vi "HFRR ADV v038.vi"() -> ()   [LabVIEW 2025] (continued)
        n794 = property on="Tab Control 5" class="TabCtl (strict)"("Value"=enum32{"OK", "NG"}."NG" ("Tab Control 5")) -> ()  [unwired: 2 in, 2 out]
      }
      frame True {
        n795 = property on="Accept & Save" class="Bool (strict)"("DisabledEnum"=T19."Enabled" ("Disabled")) -> ()  [unwired: 2 in, 2 out]
        n796 = property on="Tab Control 5" class="TabCtl (strict)"("Value"=enum32{"OK", "NG"}."OK" ("Tab Control 5")) -> ()  [unwired: 2 in, 2 out]
      }
    }
    n797 = local read "Quit"() -> (w735:bool)
  }
  n798 = while {
    shift-right: [w815] -> _
    shift-left: "Enum - Selector" -> [w816]
    stop <- w817 stop-if-true
    # "Auto Start Logic Loop"
    n799 = case shown="\"close\"" w816 {
      tunnel: [w820 w826 w853 w885 w915 Auto_Start_enum."Exit" ("Enum - Selector") Auto_Start_enum."Init" ("Enum - Selector")] -> w815
      frame "Init", Default {
        n800 = local read "Auto Start Test"() -> (w819:bool)
        n801 = Select(t=Auto_Start_enum."Humidity & Temperature On" ("Enum - Selector"), s=w819, f=Auto_Start_enum."Init") -> (s? t:f=w820:T15)
      }
      frame "Humidity & Temperature On" {
        n802 = stacked-sequence {
          tunnel: [_ _ _ _ _ _ Auto_Start_enum."Reach point" ("Enum - Selector")] -> w823
          frame #0 {
            w828 = T19."Disabled and Grayed Out" ("Disabled")
            w829 = TRUE ("Heater Button")
            n803 = property on="Humidity" class="Bool (strict)"("DisabledEnum"=w828) -> ()  [unwired: 2 in, 2 out]
            n804 = property on="Heater Button" class="Bool (strict)"("DisabledEnum"=w828) -> ()  [unwired: 2 in, 2 out]
            n805 = local write "Heater Button"(w829) -> ()
            n806 = local write "Humidity"(w829) -> ()
            n807 = property on="Heater Button" class="Bool (strict)"("Val(Sgnl)"=TRUE ("Value (Signaling)")) -> ()  [unwired: 2 in, 2 out]
          }
          frame #1 {
            n808 = Wait (ms)(milliseconds to wait=u32 3000) -> ()  [unwired: 1 out]
          }
          frame #2 {
            n809 = local read "Set Temp"() -> (w835:dbl)
            n810 = Number To Fractional String(number=w835, precision (6)=i16 2) -> (F-format string=w832:string)  [unwired: 2 in]
            n811 = Concatenate Strings("ST;" ("Command"), w832) -> (w833:string)
            n812 = local write "Due Write"(w833) -> ()
          }
          frame #3 {
            n813 = Wait (ms)(milliseconds to wait=u32 1500) -> ()  [unwired: 1 out]
          }
          frame #4 {
            (unwired) i16 2 ("precision (6)")
            n814 = local read "WriteHumidity"() -> (w837:string[])
            n815 = local read "Set Rh"() -> (w840:dbl)
            n816 = Number To Fractional String(number=w840) -> (F-format string=w841:string)  [unwired: 3 in]
            n817 = Concatenate Strings("M;" ("new element/subarray"), w841) -> (w842:string)
            n818 = Insert Into Array(array=w837, new element=w842) -> (w838:string[])  [unwired: 1 in]
            n819 = local write "WriteHumidity"(w838) -> ()
            n820 = local write "Due Write"("HE;1" ("Command")) -> ()
          }
          frame #5 {
            n821 = Wait (ms)(milliseconds to wait=u32 1500) -> ()  [unwired: 1 out]
          }
          frame #6 {
            w845 = TRUE ("Reach point temp")
            n822 = local write "Reach point Humidity"(w845) -> ()
            n823 = local write "Reach point temp"(w845) -> ()
          }
        }
        n824 = local read "Auto Start Test"() -> (w825:bool)
        n825 = Not(x=w825) -> (.not. x?=w824:bool)
        n826 = Select(t=Auto_Start_enum."close", s=w824, f=w823) -> (s? t:f=w826:T15)
      }
      frame "Reach point" {
        w854 = TRUE ("PAUSE")
        w862 = 1.0 ("y")
        w865 = 1.0 ("y")
        n827 = local read "Set Temp"() -> (w847:dbl)
        n828 = local read "Set Humidity:"() -> (w861:dbl)
        n829 = local read "Humidity ( %RH )"() -> (w866:dbl)
        n830 = Add(x=w847, y=w865) -> (x+y=w864:dbl)
        n831 = Subtract(x=w847, y=w865) -> (x-y=w863:dbl)
        n832 = Add(x=w861, y=w862) -> (x+y=w860:dbl)
        n833 = Subtract(x=w861, y=w862) -> (x-y=w859:dbl)
        n834 = local read "TEMP"() -> (w867:dbl)
        n835 = In Range and Coerce(upper limit=w860, x=w866, lower limit=w859) -> (In Range?=w848:bool)  [unwired: 1 out]
        n836 = In Range and Coerce(upper limit=w864, x=w867, lower limit=w863) -> (In Range?=w849:bool)  [unwired: 1 out]
        n837 = case shown="True" w848 {
          frame False {
          }
          frame True {
            n838 = case shown="True" "Reach point Humidity" {
              selector: "Reach point Humidity" -> [_ w873]
              frame False {
              }
              frame True {
                n839 = local read "EVENT LOG"() -> (w870:string)
                n840 = Not(x=w873) -> (.not. x?=w872:bool)
                n841 = local write "Reach point Humidity"(w872) -> ()
                n842 = call "Event Log.vi"("Content"="Target Humidity reached", "EVENT LOG"=w870) -> ("EVENT LOG"=w871:string)  [unwired: 8 in, 1 out]
                n843 = local write "EVENT LOG"(w871) -> ()
              }
            }
          }
        }
        n844 = case shown="True" w849 {
          frame False {
          }
          frame True {
            n845 = case shown="True" "Reach point temp" {
              selector: "Reach point temp" -> [_ w879]
              frame False {
              }
              frame True {
                n846 = local read "EVENT LOG"() -> (w876:string)
                n847 = Not(x=w879) -> (.not. x?=w878:bool)
                n848 = local write "Reach point temp"(w878) -> ()
                n849 = call "Event Log.vi"("Content"="Target Temperature reached", "EVENT LOG"=w876) -> ("EVENT LOG"=w877:string)  [unwired: 8 in, 1 out]
                n850 = local write "EVENT LOG"(w877) -> ()
              }
            }
          }
        }
        n851 = local read "Auto Start Test"() -> (w852:bool)
        n852 = And(x=w849, y=w848) -> (x .and. y?=w858:bool)
        n853 = Select(t=Auto_Start_enum."Maintain Stage" ("Enum - Selector"), s=w858, f=Auto_Start_enum."Reach point" ("Enum - Selector")) -> (s? t:f=w855:T15)
        n854 = Not(x=w852) -> (.not. x?=w851:bool)
        n855 = Select(t=Auto_Start_enum."close", s=w851, f=w855) -> (s? t:f=w853:T15)
        n856 = call "ELAPSED TIMER VI.vi"("RESET"=w854, "PAUSE"=w854) -> ()  [unwired: 7 in, 3 out]
      }
      frame "Maintain Stage" {
        w894 = 2.0 ("y")
        w893 = 1.0 ("y")
        # "Humidity and  temperatures Set Point  have been reached"
        n857 = local read "Set Temp"() -> (w880:dbl)
        n858 = local read "Set Humidity:"() -> (w897:dbl)
        n859 = local read "Humidity ( %RH )"() -> (w900:dbl)
        n860 = Add(x=w880, y=w893) -> (x+y=w899:dbl)
        n861 = Subtract(x=w880, y=w893) -> (x-y=w898:dbl)
        n862 = local read "TEMP"() -> (w901:dbl)
        n863 = Add(x=w897, y=w894) -> (x+y=w896:dbl)
        n864 = Subtract(x=w897, y=w894) -> (x-y=w895:dbl)
        n865 = In Range and Coerce(upper limit=w899, x=w901, lower limit=w898) -> (In Range?=w892:bool)  [unwired: 1 out]
        n866 = In Range and Coerce(upper limit=w896, x=w900, lower limit=w895) -> (In Range?=w891:bool)  [unwired: 1 out]
        n867 = And(x=w892, y=w891) -> (x .and. y?=w890:bool)
        n868 = Not(x=w890) -> (.not. x?=w889:bool)
        n869 = call "ELAPSED TIMER VI.vi"("TARGET"=60.0, "RESET"=w889, "PAUSE"=FALSE) -> ("ELAPSED INDICATION"=w886:bool)  [unwired: 6 in, 2 out]
        n870 = case shown="True" w886 {
          tunnel: w886 -> [_ w904]
          tunnel: [Auto_Start_enum."Maintain Stage" ("Enum - Selector") w903] -> w884
          frame False {
          }
          frame True {
            n871 = stacked-sequence {
              tunnel: w904 -> [_ _ _ _ _]
              tunnel: [_ _ _ _ Auto_Start_enum."Start Stage" ("Enum - Selector")] -> w903
              frame #0 {
                n872 = local read "EVENT LOG"() -> (w906:string)
                n873 = call "Event Log.vi"("Content"="Humidity and temperature set point has stabilized.", "EVENT LOG"=w906) -> ("EVENT LOG"=w907:string)  [unwired: 8 in, 1 out]
                n874 = local write "EVENT LOG"(w907) -> ()
              }
              frame #1 {
                n875 = Wait (ms)(milliseconds to wait=u32 100) -> ()  [unwired: 1 out]
              }
              frame #2 {
                n876 = local read "EVENT LOG"() -> (w910:string)
                n877 = call "Event Log.vi"("Content"="Auto Test Started", "EVENT LOG"=w910) -> ("EVENT LOG"=w911:string)  [unwired: 8 in, 1 out]
                n878 = local write "EVENT LOG"(w911) -> ()
              }
              frame #3 {
                w912 = TRUE ("RUN")
                n879 = local write "RUN"(w912) -> ()
                n880 = property on="Auto Start Temp" class="Bool (strict)"("Val(Sgnl)"=w912) -> ()  [unwired: 2 in, 2 out]
                "Auto Start Temp" <- w912
              }
              frame #4 {
              }
            }
          }
        }
        n881 = local read "Auto Start Test"() -> (w883:bool)
        n882 = Not(x=w883) -> (.not. x?=w882:bool)
        n883 = Select(t=Auto_Start_enum."close", s=w882, f=w884) -> (s? t:f=w885:T15)
      }
      frame "Start Stage" {
        w914 = TRUE ("PAUSE")
        n884 = local read "Auto Start Test"() -> (w919:bool)
        n885 = Not(x=w919) -> (.not. x?=w918:bool)
        n886 = Select(t=Auto_Start_enum."close" ("Enum - Selector"), s=w918, f=Auto_Start_enum."Start Stage" ("Enum - Selector")) -> (s? t:f=w915:T15)
        n887 = call "ELAPSED TIMER VI.vi"("RESET"=w914, "PAUSE"=w914) -> ()  [unwired: 7 in, 3 out]
      }
      frame "close" {
        w922 = FALSE ("Heater Button")
        n888 = local write "RUN"(w922) -> ()
        n889 = local write "Heater Button"(w922) -> ()
        n890 = local write "Humidity"(w922) -> ()
        n891 = local write "Auto Start Test"(w922) -> ()
        n892 = property on="Heater Button" class="Bool (strict)"("Val(Sgnl)"=FALSE ("Value (Signaling)")) -> ()  [unwired: 2 in, 2 out]
        n893 = local write "Humidity"(TRUE ("Humidity")) -> ()
      }
      frame "Exit" {
      }
    }
    n894 = Wait (ms)(milliseconds to wait=u32 100) -> ()  [unwired: 1 out]
    n895 = local read "Quit"() -> (w817:bool)
  }
  n896 = property on="Service Password Log" class="Str"("Visible"=w21) -> ()  [unwired: 2 in, 2 out]
  n897 = property on="Password 3" class="Clust (strict)"("Visible"=w21) -> ()  [unwired: 2 in, 2 out]
  n898 = while {
    stop <- w951 stop-if-true
    w934 = errorcluster {"status"=FALSE, "code"=0, "source"=""} ("error in (no error) 3")
    # "this loop is for manual report generation"
    n899 = local read "Confirm Measrurement"() -> (w933:bool)
    n900 = case shown="True" w933 {
      selector: w933 -> [_ w1041]
      tunnel: errorcluster {"status"=FALSE, "code"=0, "source"=""} ("error in (no error) 3") -> [_ w1042]
      tunnel: [_ w1040] -> _
      frame False {
      }
      frame True {
        n901 = stacked-sequence {
          tunnel: w1042 -> [_ w1075 _]
          tunnel: w1041 -> [_ _ w1182]
          tunnel: [_ w1063 _] -> w1040
          frame #0 {
            n902 = String To Path(string="C:\\LAB-IQ\\Image Calibrate v01.dcf") -> (path=w1045:path)
            n903 = Open/Create/Replace File ("Open File")(file path (use dialog)=w1045) -> (refnum out=w1046:refnum<file>)  [unwired: 5 in, 2 out]
            n904 = for {
              N: 4 -> [_]
              tunnel: w1046 -> [w1052]
              i -> [w1048]
              n905 = Read from Text File ("Read File")(file (use dialog)=w1052) -> (text=w1053:string)  [unwired: 3 in, 3 out]
              n906 = String Subset(string=w1053, offset (0)=6, length (rest)=10 ("length (rest)")) -> (substring=w1049:string)
              n907 = Fract/Exp String To Number(string=w1049) -> (number=w1047:dbl)  [unwired: 3 in, 1 out]
              n908 = case shown="3" w1048 {
                tunnel: w1047 -> [w1054 w1055 _ w1056 _]
                frame 0 {
                  n909 = local write "5x Gain"(w1054) -> ()
                }
                frame 1 {
                  n910 = local write "10x Gain"(w1055) -> ()
                }
                frame 2 {
                }
                frame 3 {
                  n911 = local write "100x gain"(w1056) -> ()
                }
                frame 4, Default {
                }
              }
            }
          }
          frame #1 {
            n912 = local read "TEST STANDARD"() -> (w1058:T3)
            n913 = case shown="\"ISO 12156\"" w1058 {
              tunnel: ["ASTM D6079" "ISO 12156"] -> w1057
              frame "ASTM D6079", Default {
              }
              frame "ISO 12156" {
              }
            }
            n914 = call "IMAGE ANALYSIS.vi"("Enum"=POST_ANALYSIS_ENUM."GET MEASUREMENTS", "error in"=w1075) -> ("error out"=w1082:errorcluster)  [unwired: 8 in, 1 out]
            n915 = local read "Magnification :"() -> (w1068:string)
            n916 = call "Stall Data Flow.vim"("value in"=w1082, "milliseconds to wait"=u32 1000) -> ("value out"=w1081:errorcluster)  [unwired: 1 out]
            n917 = local read "Test File List :"() -> (w1079:string)
            n918 = case shown="\"10x\"" w1068 {
              tunnel: [w1118 w1119] -> w1066
              frame "5x", Default {
                n919 = local read "5x Gain"() -> (w1118:dbl)
              }
              frame "10x" {
                # "5x"
                n920 = local read "10x Gain"() -> (w1119:dbl)
              }
            }
            n921 = call "IMAGE ANALYSIS.vi"("Enum"=POST_ANALYSIS_ENUM."READ", "error in"=w1081) -> ("error out"=w1078:errorcluster, "data out"=w1069:string)  [unwired: 8 in]
            n922 = Match Pattern(string=w1069, regular expression="\"type\": ") -> (after substring=w1073:string)  [unwired: 1 in, 3 out]
            n923 = call "IMAGE PATH CREATION PY.vi"("error in (no error)"=w1078, "File Name :"=w1079) -> ("error out"=w1077:errorcluster, "File Path"=w1065:path, "File Path String:"=w1060:string)  [unwired: 7 in]
            n924 = Match Pattern(string=w1073, regular expression=",") -> (before substring=w1059:string)  [unwired: 1 in, 3 out]
            n925 = local read "Calibration Tab"() -> (w1062:enum32{"Measrument", "Calibrate"})
            n926 = call "Stall Data Flow.vim"("value in"=w1077, "milliseconds to wait"=u32 250) -> ("value out"=w1061:errorcluster)  [unwired: 1 out]
            n927 = Equal?(x=w1059, y="\"rectangle\"") -> (x = y?=w1070:bool)
            n928 = case shown="False" w1070 {
              tunnel: w1069 -> [w1124 w1179]
              tunnel: w1066 -> [_ w1170]
              tunnel: cluster{"major":dbl, "minor":dbl, "average":dbl} {"major"=0.0, "minor"=0.0, "average"=0.0} -> [w1122 w1166]
              tunnel: [w1121 w1163] -> w1064
              tunnel: w1059 -> [w1123 _]
              tunnel: w1066 -> [w1120 _]
              frame False {
                n929 = Equal?(x=w1123, y="\"line\"") -> (x = y?=w1125:bool)
                n930 = case shown="True" w1125 {
                  tunnel: w1124 -> [_ w1140]
                  tunnel: w1122 -> [w1127 w1139]
                  tunnel: [w1127 w1137] -> w1121
                  tunnel: w1120 -> [_ w1136]
                  frame False {
                  }
                  frame True {
                    w1135 = 0.0 ("Major Axis")
                    n931 = Match Pattern(string=w1140, regular expression="\"length_px\":") -> (after substring=w1138:string)  [unwired: 1 in, 3 out]
                    n932 = property on="Major Axis" class="DigNum (strict)"("Caption.Text"="") -> ()  [unwired: 2 in, 2 out]
                    n933 = property on="Minor Axis" class="DigNum (strict)"("Caption.Text"="") -> ()  [unwired: 2 in, 2 out]
                    n934 = property on="Average" class="DigNum (strict)"("Caption.Text"="Line") -> ()  [unwired: 2 in, 2 out]
                    n935 = Fract/Exp String To Number(string=w1138, default (0 dbl)=0.0 ("default (0 DBL)")) -> (number=w1134:dbl)  [unwired: 2 in, 1 out]
                    "Pixel Value" <- w1134
                    n936 = Multiply(x=w1134, y=w1136) -> (x*y=w1147:dbl)
                    n937 = Multiply(x=w1147, y=1000.0) -> (x*y=w1130:dbl)
                    n938 = Divide(x=w1130, y=1000.0) -> (x/y=w1133:dbl)
                    n939 = local write "Measurment (mm)"(w1133) -> ()
                    n940 = Bundle By Name(cluster=w1139, "average"=w1130) -> (w1137:cluster{"major":dbl, "minor":dbl, "average":dbl})
                    n941 = Number To Fractional String(number=w1130, precision (6)=i16 1) -> (F-format string=w1129:string)  [unwired: 2 in]
                    n942 = local write "Minor Axis"(w1135) -> ()
                    n943 = local write "Major Axis"(w1135) -> ()
                    n944 = Fract/Exp String To Number(string=w1129) -> (number=w1128:dbl)  [unwired: 3 in, 1 out]
                    n945 = local write "Average"(w1128) -> ()
                  }
                }
              }
              frame True {
                w1167 = 1000.0 ("y")
                w1173 = 0.0 ("default (0 DBL)")
                n946 = Match Pattern(string=w1179, regular expression=" \"width_px\":") -> (after substring=w1177:string)  [unwired: 1 in, 3 out]
                n947 = Match Pattern(string=w1177, regular expression="\"height_px\":") -> (before substring=w1175:string, after substring=w1174:string)  [unwired: 1 in, 2 out]
                n948 = Fract/Exp String To Number(string=w1175, default (0 dbl)=w1173) -> (number=w1172:dbl)  [unwired: 2 in, 1 out]
                n949 = Fract/Exp String To Number(string=w1174, default (0 dbl)=w1173) -> (number=w1171:dbl)  [unwired: 2 in, 1 out]
                n950 = Multiply(x=w1172, y=w1170) -> (x*y=w1169:dbl)
                n951 = Multiply(x=w1171, y=w1170) -> (x*y=w1168:dbl)
                n952 = Multiply(x=w1169, y=w1167) -> (x*y=w1153:dbl)
                n953 = Multiply(x=w1168, y=w1167) -> (x*y=w1151:dbl)
                n954 = Add(x=w1153, y=w1151) -> (x+y=w1165:dbl)
                n955 = property on="Major Axis" class="DigNum (strict)"("Caption.Text"="Major Axis") -> ()  [unwired: 2 in, 2 out]
                n956 = property on="Minor Axis" class="DigNum (strict)"("Caption.Text"="Minor Axis") -> ()  [unwired: 2 in, 2 out]
                n957 = property on="Average" class="DigNum (strict)"("Caption.Text"="Average") -> ()  [unwired: 2 in, 2 out]
                n958 = Divide(x=w1165, y=2.0) -> (x/y=w1149:dbl)
                n959 = Bundle By Name(cluster=w1166, "major"=w1153, "minor"=w1151, "average"=w1149) -> (w1163:cluster{"major":dbl, "minor":dbl, "average":dbl})
                n960 = Number To Fractional String(number=w1151, precision (6)=i16 1) -> (F-format string=w1158:string)  [unwired: 2 in]
                n961 = Number To Fractional String(number=w1149, precision (6)=i16 1) -> (F-format string=w1159:string)  [unwired: 2 in]
                n962 = Number To Fractional String(number=w1153, precision (6)=i16 1) -> (F-format string=w1157:string)  [unwired: 2 in]
                n963 = Fract/Exp String To Number(string=w1158) -> (number=w1150:dbl)  [unwired: 3 in, 1 out]
                n964 = Fract/Exp String To Number(string=w1159) -> (number=w1148:dbl)  [unwired: 3 in, 1 out]
                n965 = Fract/Exp String To Number(string=w1157) -> (number=w1152:dbl)  [unwired: 3 in, 1 out]
                n966 = local write "Major Axis"(w1152) -> ()
                n967 = local write "Average"(w1148) -> ()
                n968 = local write "Minor Axis"(w1150) -> ()
              }
            }
            n969 = case shown="\"Measrument\", Default" w1062 {
              tunnel: w1065 -> [w1092 _]
              tunnel: w1064 -> [w1091 _]
              tunnel: [w1088 w1117] -> w1063
              tunnel: w1061 -> [w1090 w1117]
              tunnel: w1060 -> [w1089 _]
              tunnel: w1057 -> [w1087 _]
              frame "Measrument", Default {
                n970 = stacked-sequence {
                  tunnel: w1092 -> [w1110 _]
                  tunnel: w1091 -> [w1108 _]
                  tunnel: w1090 -> [w1106 _]
                  tunnel: w1089 -> [w1105 _]
                  tunnel: [w1100 _] -> w1088
                  tunnel: w1087 -> [w1093 _]
                  frame #0 {
                    n971 = call "IMAGE ANALYSIS.vi"("Enum"=POST_ANALYSIS_ENUM."SAVE IMAGE", "error in"=w1106, "IMAGE FILE PATH"=w1105) -> ("error out"=w1104:errorcluster)  [unwired: 7 in, 1 out]
                    n972 = call "Stall Data Flow.vim"("value in"=w1104, "milliseconds to wait"=u32 1000) -> ("value out"=w1095:errorcluster)  [unwired: 1 out]
                    n973 = local read "Test File List :"() -> (w1112:string)
                    n974 = call "IMAGE ANALYSIS.vi"("Enum"=POST_ANALYSIS_ENUM."MINIMIZE UI", "error in"=w1095) -> ("error out"=w1102:errorcluster)  [unwired: 8 in, 1 out]
                    n975 = Bundle By Name(cluster=T27 {"File Name"="", "Test Method"="", "Operator"="", "Fuel Description"="", "Date and time"=""} ("Main Ref"), "Test Method"=w1093, "File Name"=w1112) -> (w1113:T27)
                    n976 = call "Stall Data Flow.vim"("value in"=w1102, "milliseconds to wait"=u32 1500) -> ("value out"=w1097:errorcluster)  [unwired: 1 out]
                    n977 = call "duf file read.vi"("error in (no error)"=w1097, "Main Ref"=w1113) -> ("error out"=w1111:errorcluster, "Main Ref 2"=w1109:T27)  [unwired: 8 in]
                    n978 = call "DETECTION REPORT for manual.vi"("error in (no error)"=w1111, "return value 3"=w1108, "Image File Path"=w1110, "Main Ref"=w1109) -> ("error out"=w1107:errorcluster)  [unwired: 7 in]
                    n979 = call <vilib>:"Clear Errors.vi"("error in (no error)"=w1107) -> ("error out"=w1098:errorcluster)  [unwired: 5 in, 1 out]
                    n980 = call "IMAGE ANALYSIS.vi"("Enum"=POST_ANALYSIS_ENUM."MINIMIZE UI", "error in"=w1098) -> ("error out"=w1100:errorcluster)  [unwired: 8 in, 1 out]
                  }
                  frame #1 {
                    n981 = local write "Main Tab"(T2."HOME" ("Main Tab")) -> ()
                    n982 = local write "Main Dashboard Buttons"(T1."Home" ("Main Dashboard Buttons")) -> ()
                  }
                }
              }
              frame "Calibrate" {
              }
            }
          }
          frame #2 {
            n983 = Not(x=w1182) -> (.not. x?=w1181:bool)
            n984 = local write "Confirm Measrurement"(w1181) -> ()
            n985 = local read "Calibration Tab"() -> (w1180:enum32{"Measrument", "Calibrate"})
            n986 = case shown="\"Measrument\", Default" w1180 {
              frame "Measrument", Default {
                (unwired) T21."HOME" ("Main Tab")
                n987 = local write "Main Tab"(T2."HOME" ("Main Tab")) -> ()
              }
              frame "Calibrate" {
              }
            }
          }
        }
      }
    }
    n988 = local read "Humidity"() -> (w925:bool)
    n989 = local read "Save Change"() -> (w930:bool)
    n990 = local read "Calibrate"() -> (w931:bool)
    n991 = local read "Auto Start Test"() -> (w926:bool)
    n992 = case shown="True" w931 {
      selector: w931 -> [_ w1038]
      frame False {
      }
      frame True {
        n993 = Not(x=w1038) -> (.not. x?=w1037:bool)
        n994 = local write "Calibrate"(w1037) -> ()
        n995 = local write "Calibration Tab"(enum32{"Measrument", "Calibrate"}."Calibrate" ("Calibration Tab")) -> ()
      }
    }
    n996 = case shown="True" w930 {
      selector: w930 -> [_ w982]
      frame False {
      }
      frame True {
        n997 = stacked-sequence {
          tunnel: w982 -> [_ _ _ _ w1036]
          frame #0 {
            n998 = call "IMAGE ANALYSIS.vi"("Enum"=POST_ANALYSIS_ENUM."HIDE UI") -> ()  [unwired: 9 in, 2 out]
          }
          frame #1 {
            n999 = local read "100x gain"() -> (w984:dbl)
            n1000 = local read "10x Gain"() -> (w985:dbl)
            n1001 = local read "5x Gain"() -> (w986:dbl)
            n1002 = Number To Fractional String(number=w985, width (-)=i16 4, precision (6)=i16 7) -> (F-format string=w1007:string)  [unwired: 1 in]
            n1003 = Number To Fractional String(number=0.0, width (-)=i16 4, precision (6)=i16 7) -> (F-format string=w1002:string)  [unwired: 1 in]
            n1004 = Number To Fractional String(number=w984, width (-)=i16 4, precision (6)=i16 7) -> (F-format string=w990:string)  [unwired: 1 in]
            n1005 = Number To Fractional String(number=w986, width (-)=i16 10 ("precision (6)"), precision (6)=i16 7) -> (F-format string=w1016:string)  [unwired: 1 in]
            n1006 = Concatenate Strings("[CH1]" ("string"), w1016, " - 5x Gain" ("string"), "\r") -> (w1006:string)
            n1007 = Concatenate Strings("[CH2]" ("string"), w1007, " - 10x Gain" ("string"), "\r") -> (w1005:string)
            n1008 = Concatenate Strings("[CH3]" ("string"), w1002, " - 20x Gain" ("string"), "\r") -> (w996:string)
            n1009 = Concatenate Strings("[CH4]" ("string"), w990, " - 100x Gain" ("string"), "\r") -> (w989:string)
            n1010 = String To Path(string="C:\\LAB-IQ\\Image Calibrate v01.dcf") -> (path=w1019:path)
            n1011 = Concatenate Strings(w1006, w1005, w996, w989) -> (w1004:string)
            n1012 = call <vilib>:"Write Characters To File.vi"("append to file? (new file:F)"=FALSE, "character string"=w1004, "file path (dialog if empty)"=w1019) -> ()  [unwired: 2 in, 1 out]
          }
          frame #2 {
            n1013 = String To Path(string="C:\\LAB-IQ\\Image Calibrate v01.dcf") -> (path=w1022:path)
            n1014 = Open/Create/Replace File ("Open File")(file path (use dialog)=w1022) -> (refnum out=w1023:refnum<file>)  [unwired: 5 in, 2 out]
            n1015 = for {
              N: 4 -> [_]
              tunnel: w1023 -> [w1029]
              i -> [w1025]
              n1016 = Read from Text File ("Read File")(file (use dialog)=w1029) -> (text=w1030:string)  [unwired: 3 in, 3 out]
              n1017 = String Subset(string=w1030, offset (0)=6, length (rest)=10 ("length (rest)")) -> (substring=w1026:string)
              n1018 = Fract/Exp String To Number(string=w1026) -> (number=w1024:dbl)  [unwired: 3 in, 1 out]
              n1019 = case shown="3" w1025 {
                tunnel: w1024 -> [w1031 w1032 _ w1033 _]
                frame 0 {
                  n1020 = local write "5x Gain"(w1031) -> ()
                }
                frame 1 {
                  n1021 = local write "10x Gain"(w1032) -> ()
                }
                frame 2 {
                }
                frame 3 {
                  n1022 = local write "100x gain"(w1033) -> ()
                }
                frame 4, Default {
                }
              }
            }
          }
          frame #3 {
            n1023 = call "IMAGE ANALYSIS.vi"("Enum"=POST_ANALYSIS_ENUM."SHOW UI") -> ()  [unwired: 9 in, 2 out]
          }
          frame #4 {
            n1024 = Not(x=w1036) -> (.not. x?=w1035:bool)
            n1025 = local write "Save Change"(w1035) -> ()
          }
        }
      }
    }
    n1026 = case shown="False" w926 {
      tunnel: w925 -> [w952 _]
      frame False {
        n1027 = case shown="True" w952 {
          frame False {
          }
          frame True {
            n1028 = local read "Set Humidity:"() -> (w956:dbl)
            n1029 = local read "Set Humidity:"() -> (w959:dbl)
            n1030 = local read "Humidity ( %RH )"() -> (w960:dbl)
            n1031 = Subtract(x=w956, y=2.0) -> (x-y=w954:dbl)
            n1032 = Add(x=w959, y=2.0) -> (x+y=w955:dbl)
            n1033 = In Range and Coerce(upper limit=w955, x=w960, lower limit=w954) -> (In Range?=w953:bool)  [unwired: 1 out]
            n1034 = case shown="True" w953 {
              frame False {
              }
              frame True {
                n1035 = case shown="True" "Manual Humididty Reached" {
                  selector: "Manual Humididty Reached" -> [_ w963]
                  frame False {
                  }
                  frame True {
                    n1036 = Not(x=w963) -> (.not. x?=w962:bool)
                    n1037 = local write "Manual Humididty Reached"(w962) -> ()
                    n1038 = local read "EVENT LOG"() -> (w965:string)
                    n1039 = call "Event Log.vi"("Content"="Target Humidity reached", "EVENT LOG"=w965) -> ("EVENT LOG"=w964:string)  [unwired: 8 in, 1 out]
                    n1040 = local write "EVENT LOG"(w964) -> ()
                  }
                }
              }
            }
          }
        }
      }
      frame True {
        n1041 = local write "Manual Humididty Reached"(TRUE ("Manual Humididty Reached")) -> ()
      }
    }
    n1042 = local read "Cap Live Image"() -> (w946:bool)
    n1043 = local read "SCAR MEASURMENT"() -> (w949:enum32{"Auto Scar", "Manual Scar"})
    n1044 = Equal?(x=w949, y=enum32{"Auto Scar", "Manual Scar"}."Manual Scar" ("SCAR MEASURMENT")) -> (x = y?=w947:bool)
    n1045 = And(x=w947, y=w946) -> (x .and. y?=w945:bool)
    n1046 = Wait (ms)(milliseconds to wait=u32 250) -> ()  [unwired: 1 out]
    n1047 = case shown="True" w945 {
      selector: w945 -> [_ w1268]
      frame False {
      }
      frame True {
        n1048 = stacked-sequence {
          tunnel: [_ _ _ w1287 _] -> _
          tunnel: w1268 -> [_ _ _ _ w1294]
          frame #0 {
            w1269 = 0.0
            n1049 = local write "Major Axis"(w1269) -> ()
            n1050 = local write "Minor Axis"(w1269) -> ()
            n1051 = local write "Average"(w1269) -> ()
          }
          frame #1 {
            n1052 = call "CAMERA LIVE FEED FGV.vi"("Enum - Menu"=CAMERA_LIVE_FEED_ENUM."CAMERA MINIMIZE") -> ()  [unwired: 9 in, 2 out]
          }
          frame #2 {
            n1053 = local read "Magnification len live scar"() -> (w1273:string)
            n1054 = case shown="\"10x\", Default" w1273 {
              tunnel: ["_10x" "_5x"] -> w1272
              frame "10x", Default {
              }
              frame "5x" {
              }
            }
            n1055 = local read "FILE 3"() -> (w1279:string)
            n1056 = call <vilib>:"Trim Whitespace.vi"("string"="C:\\LAB-IQ\\images\\") -> ("trimmed string"=w1281:string)  [unwired: 1 in]
            n1057 = String To Path(string=w1281) -> (path=w1280:path)
            n1058 = Concatenate Strings(w1279, w1272, ".png" ("string")) -> (w1278:string)
            n1059 = Build Path(base path=w1280, name or relative path=w1278) -> (appended path=w1277:path)
            n1060 = Path To String(path=w1277) -> (string=w1276:string)
            n1061 = call "CAMERA LIVE FEED FGV.vi"("Enum - Menu"=CAMERA_LIVE_FEED_ENUM."CAMERA SAVE", "Image Path"=w1276) -> ("error out"=w1274:errorcluster)  [unwired: 8 in, 1 out]
            n1062 = case shown="No Error" w1274 {
              frame No Error {
                n1063 = One Button Dialog(message="Image saved successfully") -> ()  [unwired: 1 in, 1 out]
              }
              frame Error {
              }
            }
          }
          frame #3 {
            n1064 = call "LIST FILE NAMES.vi"() -> ("error out"=w1289:errorcluster, "filenames"=w1286:string[])  [unwired: 10 in]
            n1065 = call "IMAGE ANALYSIS.vi"("Enum"=POST_ANALYSIS_ENUM."SHOW UI", "error in"=w1289) -> ("error out"=w1287:errorcluster)  [unwired: 8 in, 1 out]
            n1066 = property on="Test File List :" class="CmbBox"("Strings[]"=w1286) -> ()  [unwired: 2 in, 2 out]
          }
          frame #4 {
            (unwired) T26."Report" ("Main Dashboard Buttons")
            (unwired) T28."Report" ("Main Dashboard Buttons")
            n1067 = Not(x=w1294) -> (.not. x?=w1293:bool)
            n1068 = local write "Zoom Factore"(0.0 ("Zoom Factore")) -> ()
            n1069 = local write "Cap Live Image"(w1293) -> ()
            n1070 = local write "Main Tab"(T2."Adv Scar Report" ("Main Tab")) -> ()
            n1071 = property on="Cap Live Image" class="Bool (strict)"("BoolText.Text"="Capture Image" ("Boolean Text.Text")) -> ()  [unwired: 2 in, 2 out]
            n1072 = local write "Main Dashboard Buttons"(T1."Report" ("Main Dashboard Buttons")) -> ()
          }
        }
      }
    }
    n1073 = local read "change Gain"() -> (w929:bool)
    n1074 = local read "Back Square"() -> (w928:bool)
    n1075 = case shown="True" w929 {
      selector: w929 -> [_ w973]
      frame False {
      }
      frame True {
        n1076 = stacked-sequence {
          tunnel: w973 -> [_ w981]
          frame #0 {
            n1077 = local read "Actual (µm)"() -> (w977:dbl)
            n1078 = local read "Pixel Value"() -> (w976:dbl)
            n1079 = local read "Magnification :"() -> (w975:string)
            n1080 = Divide(x=w977, y=w976) -> (x/y=w974:dbl)
            n1081 = case shown="\"10x\"" w975 {
              tunnel: w974 -> [w978 w979]
              frame "10x" {
                n1082 = local write "10x Gain"(w978) -> ()
              }
              frame "5x", Default {
                n1083 = local write "5x Gain"(w979) -> ()
              }
            }
          }
          frame #1 {
            n1084 = Not(x=w981) -> (.not. x?=w980:bool)
            n1085 = local write "change Gain"(w980) -> ()
          }
        }
      }
    }
    n1086 = case shown="True" w928 {
      selector: w928 -> [_ w971]
      frame False {
      }
      frame True {
        n1087 = Not(x=w971) -> (.not. x?=w970:bool)
        n1088 = local write "Back Square"(w970) -> ()
        n1089 = local write "Calibration Tab"(enum32{"Measrument", "Calibrate"}."Measrument" ("Calibration Tab")) -> ()
      }
    }
    n1090 = local read "Rectangle Tool"() -> (w940:bool)
    n1091 = local read "Clear ROI Tool"() -> (w939:bool)
    n1092 = local read "Open Image"() -> (w944:bool)
    n1093 = local read "line tool"() -> (w941:bool)
    n1094 = local read "OUT"() -> (w942:bool)
    n1095 = local read "In"() -> (w943:bool)
    n1096 = case shown="True" w944 {
      selector: w944 -> [_ w1254]
      tunnel: [w1245 w1256] -> _
      tunnel: w934 -> [w1245 w1255]
      frame False {
      }
      frame True {
        w1249 = "_5x" ("regular expression")
        n1097 = Not(x=w1254) -> (.not. x?=w1253:bool)
        n1098 = local write "Open Image"(w1253) -> ()
        n1099 = call "IMAGE ANALYSIS.vi"("Enum"=POST_ANALYSIS_ENUM."HIDE UI", "error in"=w1255) -> ("error out"=w1263:errorcluster)  [unwired: 8 in, 1 out]
        n1100 = call <vilib>:"Clear Errors.vi"("error in (no error)"=w1263) -> ("error out"=w1246:errorcluster)  [unwired: 5 in, 1 out]
        n1101 = call "File Dialog"("start path"=path "C:/LAB-IQ/images", "error in"=w1246) -> ("selected path"=w1248:path, "error out"=w1261:errorcluster)  [unwired: 10 in, 2 out]
        "Image path  2" <- w1248
        n1102 = call <vilib>:"Clear Errors.vi"("error in (no error)"=w1261) -> ("error out"=w1260:errorcluster)  [unwired: 5 in, 1 out]
        n1103 = call "IMAGE ANALYSIS.vi"("Enum"=POST_ANALYSIS_ENUM."OPEN FILE", "error in"=w1260, "File Path"=w1248) -> ("error out"=w1259:errorcluster)  [unwired: 7 in, 1 out]
        n1104 = call <vilib>:"Clear Errors.vi"("error in (no error)"=w1259) -> ("error out"=w1258:errorcluster)  [unwired: 5 in, 1 out]
        n1105 = call "IMAGE ANALYSIS.vi"("Enum"=POST_ANALYSIS_ENUM."SHOW UI", "error in"=w1258) -> ("error out"=w1256:errorcluster)  [unwired: 8 in, 1 out]
        n1106 = local write "Zoom Factore"(100.0 ("Zoom Factore")) -> ()
        n1107 = Strip Path(path=w1248) -> (name=w1251:string)  [unwired: 1 out]
        n1108 = Match Pattern(string=w1251, regular expression=w1249) -> (match substring=w1250:string)  [unwired: 1 in, 3 out]
        n1109 = Equal?(x=w1250, y=w1249) -> (x = y?=w1247:bool)
        n1110 = case shown="False" w1247 {
          frame False {
            n1111 = local write "Magnification :"("10x" ("Magnification :")) -> ()
          }
          frame True {
            n1112 = local write "Magnification :"("5x" ("Magnification :")) -> ()
          }
        }
      }
    }
    n1113 = case shown="True" w942 {
      selector: w942 -> [_ w1230]
      tunnel: w934 -> [w1227 w1235]
      tunnel: [w1227 w1229] -> _
      frame False {
      }
      frame True {
        n1114 = Not(x=w1230) -> (.not. x?=w1228:bool)
        n1115 = local read "Zoom Factore"() -> (w1233:dbl)
        n1116 = local write "OUT"(w1228) -> ()
        n1117 = call "IMAGE ANALYSIS.vi"("Enum"=POST_ANALYSIS_ENUM."ZOOM OUT", "error in"=w1235) -> ("error out"=w1229:errorcluster)  [unwired: 8 in, 1 out]
        n1118 = Divide(x=w1233, y=1.2) -> (x/y=w1231:dbl)
        n1119 = local write "Zoom Factore"(w1231) -> ()
      }
    }
    n1120 = case shown="True" w943 {
      selector: w943 -> [_ w1239]
      tunnel: w934 -> [w1236 w1244]
      tunnel: [w1236 w1237] -> _
      frame False {
      }
      frame True {
        n1121 = Not(x=w1239) -> (.not. x?=w1238:bool)
        n1122 = local read "Zoom Factore"() -> (w1242:dbl)
        n1123 = local write "In"(w1238) -> ()
        n1124 = call "IMAGE ANALYSIS.vi"("Enum"=POST_ANALYSIS_ENUM."ZOOM IN", "error in"=w1244) -> ("error out"=w1237:errorcluster)  [unwired: 8 in, 1 out]
        n1125 = Multiply(x=w1242, y=1.2) -> (x*y=w1240:dbl)
        n1126 = local write "Zoom Factore"(w1240) -> ()
      }
    }
    n1127 = case shown="True" w939 {
      selector: w939 -> [_ w1211]
      tunnel: w934 -> [w1209 w1213]
      tunnel: [w1209 w1212] -> _
      frame False {
      }
      frame True {
        n1128 = Not(x=w1211) -> (.not. x?=w1210:bool)
        n1129 = local write "Clear ROI Tool"(w1210) -> ()
        n1130 = call "IMAGE ANALYSIS.vi"("Enum"=POST_ANALYSIS_ENUM."CLEAR ROI", "error in"=w1213) -> ("error out"=w1212:errorcluster)  [unwired: 8 in, 1 out]
      }
    }
    n1131 = case shown="True" w941 {
      selector: w941 -> [_ w1223]
      tunnel: w934 -> [w1221 w1226]
      tunnel: [w1221 w1224] -> _
      frame False {
      }
      frame True {
        n1132 = Not(x=w1223) -> (.not. x?=w1222:bool)
        n1133 = local write "line tool"(w1222) -> ()
        n1134 = call "IMAGE ANALYSIS.vi"("Enum"=POST_ANALYSIS_ENUM."DRAW LINE", "error in"=w1226) -> ("error out"=w1224:errorcluster)  [unwired: 8 in, 1 out]
      }
    }
    n1135 = case shown="True" w940 {
      selector: w940 -> [_ w1217]
      tunnel: w934 -> [w1215 w1219]
      tunnel: [w1215 w1218] -> _
      frame False {
      }
      frame True {
        n1136 = Not(x=w1217) -> (.not. x?=w1216:bool)
        n1137 = local write "Rectangle Tool"(w1216) -> ()
        n1138 = call "IMAGE ANALYSIS.vi"("Enum"=POST_ANALYSIS_ENUM."DRAW REC", "error in"=w1219) -> ("error out"=w1218:errorcluster)  [unwired: 8 in, 1 out]
      }
    }
    n1139 = local read "SCAR MEASURMENT"() -> (w927:enum32{"Auto Scar", "Manual Scar"})
    n1140 = local read "Fit to Screen Tool"() -> (w936:bool)
    n1141 = local read "Resize Tool"() -> (w935:bool)
    n1142 = case shown="\"Manual Scar\", Default" w927 {
      frame "Auto Scar" {
        n1143 = property on="Cap Live Image" class="Bool (strict)"("BoolText.Text"="Report" ("Boolean Text.Text")) -> ()  [unwired: 2 in, 2 out]
      }
      frame "Manual Scar", Default {
        n1144 = property on="Cap Live Image" class="Bool (strict)"("BoolText.Text"="Save Image" ("Boolean Text.Text")) -> ()  [unwired: 2 in, 2 out]
      }
    }
    n1145 = local read "ROI Color Tool"() -> (w937:bool)
    n1146 = local read "Pan Tool"() -> (w938:bool)
    n1147 = case shown="True" w938 {
      selector: w938 -> [_ w1205]
      tunnel: w934 -> [w1203 w1207]
      tunnel: [w1203 w1206] -> _
      frame False {
      }
      frame True {
        n1148 = Not(x=w1205) -> (.not. x?=w1204:bool)
        n1149 = call "IMAGE ANALYSIS.vi"("Enum"=POST_ANALYSIS_ENUM."PAN", "error in"=w1207) -> ("error out"=w1206:errorcluster)  [unwired: 8 in, 1 out]
        n1150 = local write "Pan Tool"(w1204) -> ()
      }
    }
    n1151 = case shown="True" w935 {
      selector: w935 -> [_ w1189]
      tunnel: w934 -> [w1184 w1186]
      tunnel: [w1184 w1185] -> _
      frame False {
      }
      frame True {
        n1152 = Not(x=w1189) -> (.not. x?=w1188:bool)
        n1153 = local write "Resize Tool"(w1188) -> ()
        n1154 = call "IMAGE ANALYSIS.vi"("Enum"=POST_ANALYSIS_ENUM."RESIZE MODE", "error in"=w1186) -> ("error out"=w1185:errorcluster)  [unwired: 8 in, 1 out]
      }
    }
    n1155 = case shown="True" w936 {
      selector: w936 -> [_ w1194]
      tunnel: [w1190 w1195] -> _
      tunnel: w934 -> [w1190 w1193]
      frame False {
      }
      frame True {
        n1156 = Not(x=w1194) -> (.not. x?=w1192:bool)
        n1157 = local write "Zoom Factore"(100.0 ("Zoom Factore")) -> ()
        n1158 = local write "Fit to Screen Tool"(w1192) -> ()
        n1159 = call "IMAGE ANALYSIS.vi"("Enum"=POST_ANALYSIS_ENUM."FIT", "error in"=w1193) -> ("error out"=w1195:errorcluster)  [unwired: 8 in, 1 out]
      }
    }
    n1160 = case shown="True" w937 {
      selector: w937 -> [_ w1200]
      tunnel: [w1197 w1201] -> _
      tunnel: w934 -> [w1197 w1198]
      frame False {
      }
      frame True {
        n1161 = Not(x=w1200) -> (.not. x?=w1199:bool)
        n1162 = local write "ROI Color Tool"(w1199) -> ()
        n1163 = call "IMAGE ANALYSIS.vi"("Enum"=POST_ANALYSIS_ENUM."SET ROI COLOR", "error in"=w1198) -> ("error out"=w1201:errorcluster)  [unwired: 8 in, 1 out]
      }
    }
    n1164 = local read "Quit"() -> (w951:bool)
  }
  n1165 = while {
    stop <- w1296 stop-if-true
    n1166 = local read "Image Path"() -> (w1299:path)
    n1167 = local read "Print 3"() -> (w1302:bool)
    n1168 = Equal?(x=w1299, y=path "") -> (x = y?=w1298:bool)
    n1169 = Not(x=w1298) -> (.not. x?=w1297:bool)
    n1170 = property on="Print 3" class="Bool (strict)"("Visible"=w1297) -> ()  [unwired: 2 in, 2 out]
    n1171 = case shown="True" w1302 {
      frame False {
        n1172 = local write "Rd"(TRUE ("Boolean 7")) -> ()
      }
      frame True {
        n1173 = flat-sequence {
          tunnel: [w1342] -> w1310
          tunnel: [w1329] -> w1308
          tunnel: [w1339] -> w1304
          tunnel: w1310 -> [w1351]
          tunnel: [w1351] -> w1309
          tunnel: w1308 -> [w1350]
          tunnel: [w1350] -> w1307
          tunnel: [w1348] -> w1306
          tunnel: [w1347] -> w1305
          tunnel: w1304 -> [w1347]
          tunnel: w1309 -> [w1353]
          tunnel: w1307 -> [w1354]
          tunnel: w1306 -> [_]
          tunnel: w1305 -> [w1352]
          frame #0 {
            n1174 = case shown="True" "Rd" {
              frame False {
              }
              frame True {
                n1175 = while {
                  tunnel: "abcdefABCDEF" ("string 2") -> [w1321]
                  shift-right: [w1319] -> w1313
                  shift-left: "" -> [w1318]
                  i -> [w1328]
                  stop <- w1327 stop-if-true
                  n1176 = Random Number (0-1)() -> (number: 0 to 1=w1322:dbl)
                  n1177 = Multiply(x=w1322, y=62.0) -> (x*y=w1324:dbl)
                  n1178 = Decrement(x="Length 2") -> (x-1=w1317:i16)
                  n1179 = To Word Integer(number=w1324) -> (16bit integer=w1325:i16)
                  n1180 = String Subset(string=w1321, offset (0)=w1325, length (rest)=1 ("length (rest)")) -> (substring=w1320:string)
                  n1181 = Greater Or Equal?(x=w1328, y=w1317) -> (x >= y?=w1327:bool)
                  n1182 = Concatenate Strings(w1320, w1318) -> (w1319:string)
                }
                "String 10" <- w1313
                n1183 = local write "Rd"(FALSE ("Boolean 7")) -> ()
              }
            }
          }
          frame #1 {
            w1340 = "_resized.jpg" ("command line")
            (unwired) ".jpg -resize 320x240 " ("string")
            (unwired) "Choose an Image File" ("prompt")
            # "-resize 1798x425"
            n1184 = local read "Image Path"() -> (w1334:path)
            n1185 = Strip Path(path=w1334) -> (stripped path=w1329:path, name=w1330:string)
            n1186 = Match Pattern(string=w1330, regular expression=".jpg") -> (before substring=→"before substring 2":string, after substring=→"after substring":string)  [unwired: 1 in, 2 out]
            n1187 = Match Pattern(string=w1330, regular expression="\\") -> (before substring=w1336:string)  [unwired: 1 in, 3 out]
            n1188 = Match Pattern(string=w1336, regular expression=".jpg") -> (before substring=w1335:string)  [unwired: 1 in, 3 out]
            n1189 = Concatenate Strings("cmd /c convert " ("string"), w1335, ".jpg -resize 320x240  " ("command line"), w1335, w1340) -> (w1343:string)
            n1190 = call <vilib>:"System Exec.vi"("run minimized? (F)"=TRUE, "wait until completion? (T)"=TRUE, "working directory"=w1329, "command line"=w1343) -> ("error out"=w1342:errorcluster)  [unwired: 4 in, 3 out]
            "error out 2" <- w1342
            n1191 = Concatenate Strings(w1335, w1340) -> (w1339:string)
          }
          frame #2 {
            n1192 = Wait (ms)(milliseconds to wait=u32 2000 ("millisecond timer value")) -> (millisecond timer value=w1348:u32)
          }
          frame #3 {
            n1193 = case shown="No Error" w1353 {
              tunnel: w1354 -> [w1357 _]
              tunnel: w1352 -> [w1355 _]
              frame No Error {
                (unwired) ".jpg" ("string")
                n1194 = Path To String(path=w1357) -> (string=w1361:string)
                n1195 = Concatenate Strings(w1361, "\\" ("string"), w1355) -> (w1360:string)
                n1196 = String To Path(string=w1360) -> (path=w1359:path)
                n1197 = call <vilib>:"Read JPEG File.vi"("path to JPEG file"=w1359) -> ("image data"=w1363:T16)  [unwired: 8 in, 2 out]
                "image data" <- w1363
                n1198 = local write "Print 3"(FALSE ("Print 2")) -> ()
                n1199 = call <vilib>:"Draw Flattened Pixmap.vi"("image data"=w1363) -> ("new picture"=→"new picture":picture)  [unwired: 8 in]
              }
              frame Error {
              }
            }
          }
        }
      }
    }
    n1200 = Wait (ms)(milliseconds to wait=u32 20 ("millisecond timer value")) -> ()  [unwired: 1 out]
    n1201 = local read "Quit"() -> (w1296:bool)
  }
  n1202 = while {
    tunnel: w38 -> [_]
    tunnel: w24 -> [_]
    stop <- w1393 stop-if-true
    # "New Adv Logics"
    n1203 = local read "Main Tab"() -> (w1374:T2)
    n1204 = local read "Main Tab"() -> (w1391:T2)
    n1205 = local read "Sign In"() -> (w1390:bool)
    n1206 = case shown="\"Adv Scar\"" w1374 {
      frame "HOME", Default {
        n1207 = local read "LIVE FEED MIN TEMP"() -> (w1526:bool)
        n1208 = local write "LIVE FEED MAX TEMP"(TRUE ("LIVE FEED MAX TEMP")) -> ()
        n1209 = local read "CAMERA ROI MIN TEMP"() -> (w1524:bool)
        n1210 = case shown="True" w1526 {
          selector: w1526 -> [_ w1533]
          frame False {
          }
          frame True {
            n1211 = Not(x=w1533) -> (.not. x?=w1532:bool)
            n1212 = local write "LIVE FEED MIN TEMP"(w1532) -> ()
            n1213 = call "CAMERA LIVE FEED FGV.vi"("Enum - Menu"=CAMERA_LIVE_FEED_ENUM."CAMERA MINIMIZE") -> ()  [unwired: 9 in, 2 out]
          }
        }
        n1214 = case shown="True" w1524 {
          selector: w1524 -> [_ w1530]
          frame False {
          }
          frame True {
            n1215 = Not(x=w1530) -> (.not. x?=w1529:bool)
            n1216 = local write "CAMERA ROI MIN TEMP"(w1529) -> ()
            n1217 = call "IMAGE ANALYSIS.vi"("Enum"=POST_ANALYSIS_ENUM."MINIMIZE UI") -> ()  [unwired: 9 in, 2 out]
          }
        }
        n1218 = local write "CAMERA ROI MAX TEMP"(TRUE ("CAMERA ROI MAX TEMP")) -> ()
      }
      frame "Test Setup" {
        n1219 = local read "LIVE FEED MIN TEMP"() -> (w1536:bool)
        n1220 = local read "CAMERA ROI MIN TEMP"() -> (w1534:bool)
        n1221 = local write "LIVE FEED MAX TEMP"(TRUE ("LIVE FEED MAX TEMP")) -> ()
        n1222 = case shown="True" w1536 {
          selector: w1536 -> [_ w1543]
          frame False {
          }
          frame True {
            n1223 = Not(x=w1543) -> (.not. x?=w1542:bool)
            n1224 = local write "LIVE FEED MIN TEMP"(w1542) -> ()
            n1225 = call "CAMERA LIVE FEED FGV.vi"("Enum - Menu"=CAMERA_LIVE_FEED_ENUM."CAMERA MINIMIZE") -> ()  [unwired: 9 in, 2 out]
          }
        }
        n1226 = case shown="True" w1534 {
          selector: w1534 -> [_ w1540]
          frame False {
          }
          frame True {
            n1227 = Not(x=w1540) -> (.not. x?=w1539:bool)
            n1228 = local write "CAMERA ROI MIN TEMP"(w1539) -> ()
            n1229 = call "IMAGE ANALYSIS.vi"("Enum"=POST_ANALYSIS_ENUM."MINIMIZE UI") -> ()  [unwired: 9 in, 2 out]
          }
        }
        n1230 = local write "CAMERA ROI MAX TEMP"(TRUE ("CAMERA ROI MAX TEMP")) -> ()
      }
      frame "Acquire" {
        n1231 = local read "LIVE FEED MIN TEMP"() -> (w1546:bool)
        n1232 = local write "LIVE FEED MAX TEMP"(TRUE ("LIVE FEED MAX TEMP")) -> ()
        n1233 = local read "CAMERA ROI MIN TEMP"() -> (w1544:bool)
        n1234 = case shown="True" w1546 {
          selector: w1546 -> [_ w1553]
          frame False {
          }
          frame True {
            n1235 = Not(x=w1553) -> (.not. x?=w1552:bool)
            n1236 = local write "LIVE FEED MIN TEMP"(w1552) -> ()
            n1237 = call "CAMERA LIVE FEED FGV.vi"("Enum - Menu"=CAMERA_LIVE_FEED_ENUM."CAMERA MINIMIZE") -> ()  [unwired: 9 in, 2 out]
          }
        }
        n1238 = case shown="True" w1544 {
          selector: w1544 -> [_ w1550]
          frame False {
          }
          frame True {
            n1239 = Not(x=w1550) -> (.not. x?=w1549:bool)
            n1240 = local write "CAMERA ROI MIN TEMP"(w1549) -> ()
            n1241 = call "IMAGE ANALYSIS.vi"("Enum"=POST_ANALYSIS_ENUM."MINIMIZE UI") -> ()  [unwired: 9 in, 2 out]
          }
        }
        n1242 = local write "CAMERA ROI MAX TEMP"(TRUE ("CAMERA ROI MAX TEMP")) -> ()
      }
      frame "Adv Scar" {
        n1243 = local read "CAMERA ROI MIN TEMP"() -> (w1554:bool)
        n1244 = case shown="True" "LIVE FEED MAX TEMP" {
          selector: "LIVE FEED MAX TEMP" -> [_ w1575]
          frame False {
          }
          frame True {
            n1245 = Not(x=w1575) -> (.not. x?=w1574:bool)
            n1246 = local write "LIVE FEED MAX TEMP"(w1574) -> ()
            n1247 = call "CAMERA LIVE FEED FGV.vi"("Enum - Menu"=CAMERA_LIVE_FEED_ENUM."CAMERA RESTORE") -> ("error out"=w1565:errorcluster)  [unwired: 9 in, 1 out]
            n1248 = Type Cast(type=30, x=0) -> (*(type *) &x=w1569:i32)
            n1249 = Add(x=w1569, y=48) -> (x+y=w1570:i32)
            n1250 = call "CAMERA LIVE FEED FGV.vi"("Enum - Menu"=CAMERA_LIVE_FEED_ENUM."CAMERA MODE SET", "error in (no error)"=w1565, "CAMERA MODE"=w1570) -> ("error out"=w1562:errorcluster)  [unwired: 7 in, 1 out]
            n1251 = call "CAMERA LIVE FEED FGV.vi"("Enum - Menu"=CAMERA_LIVE_FEED_ENUM."CAMERA GRAY", "error in (no error)"=w1562) -> ("error out"=w1561:errorcluster)  [unwired: 8 in, 1 out]
            n1252 = call "LIST FILE NAMES.vi"("error in (no error)"=w1561) -> ("error out"=w1571:errorcluster, "filenames"=w1572:string[])  [unwired: 9 in]
            n1253 = property on="FILE 3" class="CmbBox"(error in=w1571, "Strings[]"=w1572) -> ()  [unwired: 1 in, 2 out]
          }
        }
        n1254 = case shown="True" w1554 {
          selector: w1554 -> [_ w1560]
          frame False {
          }
          frame True {
            n1255 = Not(x=w1560) -> (.not. x?=w1559:bool)
            n1256 = local write "CAMERA ROI MIN TEMP"(w1559) -> ()
            n1257 = call "IMAGE ANALYSIS.vi"("Enum"=POST_ANALYSIS_ENUM."MINIMIZE UI") -> ()  [unwired: 9 in, 2 out]
          }
        }
        n1258 = local write "CAMERA ROI MAX TEMP"(TRUE ("CAMERA ROI MAX TEMP")) -> ()
        "LIVE FEED MIN TEMP" <- TRUE ("LIVE FEED MIN TEMP")
      }
      frame "Adv Scar Report" {
        n1259 = local read "CAMERA ROI MAX TEMP"() -> (w1576:bool)
        n1260 = local read "LIVE FEED MIN TEMP"() -> (w1578:bool)
        n1261 = local write "LIVE FEED MAX TEMP"(TRUE ("LIVE FEED MAX TEMP")) -> ()
        n1262 = case shown="True" w1578 {
          selector: w1578 -> [_ w1587]
          frame False {
          }
          frame True {
            n1263 = Not(x=w1587) -> (.not. x?=w1586:bool)
            n1264 = local write "LIVE FEED MIN TEMP"(w1586) -> ()
            n1265 = call "CAMERA LIVE FEED FGV.vi"("Enum - Menu"=CAMERA_LIVE_FEED_ENUM."CAMERA MINIMIZE") -> ()  [unwired: 9 in, 2 out]
          }
        }
        n1266 = case shown="True" w1576 {
          selector: w1576 -> [_ w1584]
          frame False {
          }
          frame True {
            n1267 = Not(x=w1584) -> (.not. x?=w1582:bool)
            n1268 = local write "CAMERA ROI MAX TEMP"(w1582) -> ()
            n1269 = call "IMAGE ANALYSIS.vi"("Enum"=POST_ANALYSIS_ENUM."SHOW UI") -> ("error out"=w1581:errorcluster)  [unwired: 9 in, 1 out]
            n1270 = call "LIST FILE NAMES.vi"("error in (no error)"=w1581) -> ("filenames"=w1580:string[])  [unwired: 9 in, 1 out]
            n1271 = property on="Test File List :" class="CmbBox"("Strings[]"=w1580) -> ()  [unwired: 2 in, 2 out]
          }
        }
        n1272 = local write "CAMERA ROI MIN TEMP"(TRUE ("CAMERA ROI MIN TEMP")) -> ()
      }
      frame "Compare Files" {
        n1273 = local read "LIVE FEED MIN TEMP"() -> (w1590:bool)
        n1274 = local write "LIVE FEED MAX TEMP"(TRUE ("LIVE FEED MAX TEMP")) -> ()
        n1275 = local read "CAMERA ROI MIN TEMP"() -> (w1588:bool)
        n1276 = case shown="True" w1590 {
          selector: w1590 -> [_ w1597]
          frame False {
          }
          frame True {
            n1277 = Not(x=w1597) -> (.not. x?=w1596:bool)
            n1278 = local write "LIVE FEED MIN TEMP"(w1596) -> ()
            n1279 = call "CAMERA LIVE FEED FGV.vi"("Enum - Menu"=CAMERA_LIVE_FEED_ENUM."CAMERA MINIMIZE") -> ()  [unwired: 9 in, 2 out]
          }
        }
        n1280 = case shown="True" w1588 {
          selector: w1588 -> [_ w1594]
          frame False {
          }
          frame True {
            n1281 = Not(x=w1594) -> (.not. x?=w1593:bool)
            n1282 = local write "CAMERA ROI MIN TEMP"(w1593) -> ()
            n1283 = call "IMAGE ANALYSIS.vi"("Enum"=POST_ANALYSIS_ENUM."MINIMIZE UI") -> ()  [unwired: 9 in, 2 out]
          }
        }
        n1284 = local write "CAMERA ROI MAX TEMP"(TRUE ("CAMERA ROI MAX TEMP")) -> ()
      }
      frame "About" {
        n1285 = local read "LIVE FEED MIN TEMP"() -> (w1600:bool)
        n1286 = local write "LIVE FEED MAX TEMP"(TRUE ("LIVE FEED MAX TEMP")) -> ()
        n1287 = local read "CAMERA ROI MIN TEMP"() -> (w1599:bool)
        n1288 = case shown="True" w1600 {
          selector: w1600 -> [_ w1607]
          frame False {
          }
          frame True {
            n1289 = Not(x=w1607) -> (.not. x?=w1606:bool)
            n1290 = local write "LIVE FEED MIN TEMP"(w1606) -> ()
            n1291 = call "CAMERA LIVE FEED FGV.vi"("Enum - Menu"=CAMERA_LIVE_FEED_ENUM."CAMERA MINIMIZE") -> ()  [unwired: 9 in, 2 out]
          }
        }
        n1292 = case shown="True" w1599 {
          selector: w1599 -> [_ w1604]
          frame False {
          }
          frame True {
            n1293 = Not(x=w1604) -> (.not. x?=w1603:bool)
            n1294 = local write "CAMERA ROI MIN TEMP"(w1603) -> ()
            n1295 = call "IMAGE ANALYSIS.vi"("Enum"=POST_ANALYSIS_ENUM."MINIMIZE UI") -> ()  [unwired: 9 in, 2 out]
          }
        }
        n1296 = local write "CAMERA ROI MAX TEMP"(TRUE ("CAMERA ROI MIN TEMP")) -> ()
      }
      frame "Advance" {
        n1297 = local read "LIVE FEED MIN TEMP"() -> (w1610:bool)
        n1298 = local write "LIVE FEED MAX TEMP"(TRUE ("LIVE FEED MAX TEMP")) -> ()
        n1299 = local read "CAMERA ROI MIN TEMP"() -> (w1608:bool)
        n1300 = case shown="True" w1610 {
          selector: w1610 -> [_ w1617]
          frame False {
          }
          frame True {
            n1301 = Not(x=w1617) -> (.not. x?=w1616:bool)
            n1302 = local write "LIVE FEED MIN TEMP"(w1616) -> ()
            n1303 = call "CAMERA LIVE FEED FGV.vi"("Enum - Menu"=CAMERA_LIVE_FEED_ENUM."CAMERA MINIMIZE") -> ()  [unwired: 9 in, 2 out]
          }
        }
        n1304 = local write "CAMERA ROI MAX TEMP"(TRUE ("CAMERA ROI MAX TEMP")) -> ()